vi "TLB Native Dynamic Events ver 0.26a.vi"() -> ()   [LabVIEW 2018] (continued)
              frame "Start Task 1", Default {
                # ">> T: Breaks out of state loop; F: Stays in loop>>"
                # ">> Manual override >>"
                # ">> Checks if time is up>>"
                # "Stays in Task 5D until the object is detected"
                # "T: Go back to idle, F: Continue with task\""
                # ">> Manual override >>"
                n604 = case shown="False" w1776 {
                  tunnel: [w1789 w1795] -> w1785
                  tunnel: w1777 -> [w1787 w1793]
                  frame False {
                    n605 = for {
                      tunnel: string[] ["READ STEPPER VALUES", "Y STEPPER CONTROL", ""] ("element") -> [w1790] mode=indexing
                      shift-right: [w1792] -> w1789
                      shift-left: w1787 -> [w1791]
                      n606 = Enqueue Element(queue=w1791, element=w1790) -> (queue out=w1792:refnum<queue>)  [unwired: 2 in, 2 out]
                    }
                  }
                  frame True {
                    n607 = for {
                      shift-right: [w1797] -> w1795
                      shift-left: w1793 -> [w1798]
                      tunnel: string[] ["DISPOSE BUFFERS", "READ STEPPER VALUES", ""] -> [w1796] mode=indexing
                      n608 = Enqueue Element(queue=w1798, element=w1796) -> (queue out=w1797:refnum<queue>)  [unwired: 2 in, 2 out]
                    }
                  }
                }
                n609 = Or(x=w1776, y=w1781) -> (x .or. y?=w1783:bool)
                n610 = Select(t=State_Type_Definitions,_for_0.26g_versions_and_later_2."True Stop" ("Enum"), s=w1781, f=State_Type_Definitions,_for_0.26g_versions_and_later_2."Task 8I: ARM GRAB HEIGHT" ("Enum")) -> (s? t:f=w1778:T18)
                n611 = Select(t=w1778, s=w1783, f=State_Type_Definitions,_for_0.26g_versions_and_later_2."Task 8H: ARM ADJUST" ("Enum")) -> (s? t:f=w1782:T18)
              }
              frame "Exit" {
                n612 = for {
                  shift-right: [w1805] -> w1802
                  shift-left: w1799 -> [w1806]
                  tunnel: string[] ["STOP", "RESET ENCODERS", "RESET YAW", "ARDUINO MODE 0"] -> [w1804] mode=indexing
                  n613 = Enqueue Element(queue=w1806, element=w1804) -> (queue out=w1805:refnum<queue>)  [unwired: 2 in, 2 out]
                }
              }
            }
            n614 = Bundle By Name(cluster=w1765, "yStepper desired"=w1761) -> (w1764:T20)
          }
          frame 35 {
            # ">>> Motor control cluster >>>"
            # ">>> yStepper command>>>"
            # ">> Manual override >>"
            n615 = Dequeue Element(queue=w1817, timeout in ms (-1)=w1816, error in (no error)=w1818) -> (element=w1815:T10)  [unwired: 3 out]
            n616 = Equal?(x=w1814, y=u8 1) -> (x = y?=w1812:bool)
            n617 = case shown="\"Start Task 1\", Default" w1815 {
              tunnel: [w1828 State_Type_Definitions,_for_0.26g_versions_and_later_2."True Stop" ("Enum")] -> w1819
              tunnel: [w1831 w1848] -> w1820
              tunnel: [State_Type_Definitions,_for_0.26g_versions_and_later_2."Idle" ("Enum") State_Type_Definitions,_for_0.26g_versions_and_later_2."Shutdown" ("Enum")] -> w1821
              tunnel: w1812 -> [w1827 _]
              tunnel: w1811 -> [w1826 _]
              tunnel: w1810 -> [w1822 w1845]
              frame "Start Task 1", Default {
                # "Stays in Task 5F until stepper reaches desired \nheight"
                # "T: Go back to idle, F: Continue with task\""
                # ">> Manual override >>"
                n618 = case shown="True" w1827 {
                  tunnel: [w1835 w1841] -> w1831
                  tunnel: w1822 -> [w1833 w1839]
                  frame False {
                    n619 = for {
                      tunnel: string[] ["Z STEPPER GRAB HEIGHT", "READ STEPPER VALUES"] ("element") -> [w1836] mode=indexing
                      shift-right: [w1838] -> w1835
                      shift-left: w1833 -> [w1837]
                      n620 = Enqueue Element(queue=w1837, element=w1836) -> (queue out=w1838:refnum<queue>)  [unwired: 2 in, 2 out]
                    }
                  }
                  frame True {
                    n621 = for {
                      shift-right: [w1843] -> w1841
                      shift-left: w1839 -> [w1844]
                      tunnel: string[] ["SET TIMER 2", "CLOSE CLAW", ""] -> [w1842] mode=indexing
                      n622 = Enqueue Element(queue=w1844, element=w1842) -> (queue out=w1843:refnum<queue>)  [unwired: 2 in, 2 out]
                    }
                  }
                }
                n623 = Or(x=w1827, y=w1826) -> (x .or. y?=w1829:bool)
                n624 = Select(t=State_Type_Definitions,_for_0.26g_versions_and_later_2."True Stop" ("Enum"), s=w1826, f=State_Type_Definitions,_for_0.26g_versions_and_later_2."Task 8J: CLOSE CLAW" ("Enum")) -> (s? t:f=w1823:T18)
                n625 = Select(t=w1823, s=w1829, f=State_Type_Definitions,_for_0.26g_versions_and_later_2."Task 8I: ARM GRAB HEIGHT" ("Enum")) -> (s? t:f=w1828:T18)
              }
              frame "Exit" {
                n626 = for {
                  shift-right: [w1851] -> w1848
                  shift-left: w1845 -> [w1852]
                  tunnel: string[] ["STOP", "RESET ENCODERS", "RESET YAW", "ARDUINO MODE 0"] -> [w1850] mode=indexing
                  n627 = Enqueue Element(queue=w1852, element=w1850) -> (queue out=w1851:refnum<queue>)  [unwired: 2 in, 2 out]
                }
              }
            }
          }
          frame 36 {
            # ">>> yStepper command>>>"
            # ">> Manual override >>"
            n628 = Dequeue Element(queue=w1863, timeout in ms (-1)=w1862, error in (no error)=w1861) -> (element=w1860:T10)  [unwired: 3 out]
            n629 = case shown="\"Start Task 1\", Default" w1860 {
              tunnel: [w1872 State_Type_Definitions,_for_0.26g_versions_and_later_2."True Stop" ("Enum")] -> w1865
              tunnel: [w1875 w1892] -> w1858
              tunnel: [State_Type_Definitions,_for_0.26g_versions_and_later_2."Idle" ("Enum") State_Type_Definitions,_for_0.26g_versions_and_later_2."Shutdown" ("Enum")] -> w1857
              tunnel: w1859 -> [w1866 _]
              tunnel: w1864 -> [w1871 w1889]
              tunnel: w1855 -> [w1870 _]
              frame "Start Task 1", Default {
                # ">> Is time up? >>"
                # "Determines if object is in range to pick up"
                # ">> Manual override >>"
                n630 = case shown="True" w1870 {
                  tunnel: [w1879 w1885] -> w1875
                  tunnel: w1871 -> [w1877 w1883]
                  frame False {
                    n631 = for {
                      tunnel: string[] ["CLOSE CLAW", "START TIMER"] ("element") -> [w1880] mode=indexing
                      shift-right: [w1882] -> w1879
                      shift-left: w1877 -> [w1881]
                      n632 = Enqueue Element(queue=w1881, element=w1880) -> (queue out=w1882:refnum<queue>)  [unwired: 2 in, 2 out]
                    }
                  }
                  frame True {
                    n633 = for {
                      shift-right: [w1887] -> w1885
                      shift-left: w1883 -> [w1888]
                      tunnel: string[] ["READ STEPPER VALUES", "", ""] -> [w1886] mode=indexing
                      n634 = Enqueue Element(queue=w1888, element=w1886) -> (queue out=w1887:refnum<queue>)  [unwired: 2 in, 2 out]
                    }
                  }
                }
                n635 = Or(x=w1870, y=w1866) -> (x .or. y?=w1873:bool)
                n636 = Select(t=State_Type_Definitions,_for_0.26g_versions_and_later_2."True Stop" ("Enum"), s=w1866, f=State_Type_Definitions,_for_0.26g_versions_and_later_2."Task 8K: RAISE MY SWORD" ("Enum")) -> (s? t:f=w1868:T18)
                n637 = Select(t=w1868, s=w1873, f=State_Type_Definitions,_for_0.26g_versions_and_later_2."Task 8J: CLOSE CLAW" ("Enum")) -> (s? t:f=w1872:T18)
              }
              frame "Exit" {
                n638 = for {
                  shift-right: [w1895] -> w1892
                  shift-left: w1889 -> [w1896]
                  tunnel: string[] ["STOP", "RESET ENCODERS", "RESET YAW", "ARDUINO MODE 0"] -> [w1894] mode=indexing
                  n639 = Enqueue Element(queue=w1896, element=w1894) -> (queue out=w1895:refnum<queue>)  [unwired: 2 in, 2 out]
                }
              }
            }
          }
          frame 37 {
            # ">>> yStepper command>>>"
            # ">> Manual override >>"
            n640 = Dequeue Element(queue=w1907, timeout in ms (-1)=w1906, error in (no error)=w1908) -> (element=w1905:T10)  [unwired: 3 out]
            n641 = Equal?(x=w1904, y=u8 60) -> (x = y?=w1902:bool)
            n642 = case shown="\"Start Task 1\", Default" w1905 {
              tunnel: [w1918 State_Type_Definitions,_for_0.26g_versions_and_later_2."True Stop" ("Enum")] -> w1909
              tunnel: [w1921 w1938] -> w1910
              tunnel: [State_Type_Definitions,_for_0.26g_versions_and_later_2."Idle" ("Enum") State_Type_Definitions,_for_0.26g_versions_and_later_2."Shutdown" ("Enum")] -> w1911
              tunnel: w1902 -> [w1917 _]
              tunnel: w1901 -> [w1916 _]
              tunnel: w1900 -> [w1912 w1935]
              frame "Start Task 1", Default {
                # "Stays in Task 5_A until stepper reaches desired \nheight"
                # "T: Go back to idle, F: Continue with task\""
                # ">> Manual override >>"
                n643 = case shown="True" w1917 {
                  tunnel: [w1925 w1931] -> w1921
                  tunnel: w1912 -> [w1923 w1929]
                  frame False {
                    n644 = for {
                      tunnel: string[] ["Z STEPPER CAM HEIGHT", "READ STEPPER VALUES"] ("element") -> [w1926] mode=indexing
                      shift-right: [w1928] -> w1925
                      shift-left: w1923 -> [w1927]
                      n645 = Enqueue Element(queue=w1927, element=w1926) -> (queue out=w1928:refnum<queue>)  [unwired: 2 in, 2 out]
                    }
                  }
                  frame True {
                    n646 = for {
                      shift-right: [w1933] -> w1931
                      shift-left: w1929 -> [w1934]
                      tunnel: string[] ["CAM CLOSE", "DISPOSE CAM BUFFERS", "DISPOSE PROC BUFFERS", "RESET ENCODERS"] -> [w1932] mode=indexing
                      n647 = Enqueue Element(queue=w1934, element=w1932) -> (queue out=w1933:refnum<queue>)  [unwired: 2 in, 2 out]
                    }
                  }
                }
                n648 = Or(x=w1917, y=w1916) -> (x .or. y?=w1919:bool)
                n649 = Select(t=State_Type_Definitions,_for_0.26g_versions_and_later_2."True Stop" ("Enum"), s=w1916, f=State_Type_Definitions,_for_0.26g_versions_and_later_2."True Stop" ("Enum")) -> (s? t:f=w1913:T18)
                n650 = Select(t=w1913, s=w1919, f=State_Type_Definitions,_for_0.26g_versions_and_later_2."Task 8K: RAISE MY SWORD" ("Enum")) -> (s? t:f=w1918:T18)
              }
              frame "Exit" {
                n651 = for {
                  shift-right: [w1941] -> w1938
                  shift-left: w1935 -> [w1942]
                  tunnel: string[] ["STOP", "RESET ENCODERS", "RESET YAW", "ARDUINO MODE 0"] -> [w1940] mode=indexing
                  n652 = Enqueue Element(queue=w1942, element=w1940) -> (queue out=w1941:refnum<queue>)  [unwired: 2 in, 2 out]
                }
              }
            }
          }
          frame 38 {
            # ">>> Motor control cluster >>>"
            # ">> Stepper height reeached >>"
            # ">>> yStepper command>>>"
            # ">> Manual override >>"
            n653 = Dequeue Element(queue=w1954, timeout in ms (-1)=w1949, error in (no error)=w1953) -> (element=w1957:T10)  [unwired: 3 out]
            n654 = Equal?(x=w1951, y=u8 50) -> (x = y?=w1955:bool)
            n655 = case shown="\"Start Task 1\", Default" w1957 {
              tunnel: [w1968 State_Type_Definitions,_for_0.26g_versions_and_later_2."True Stop" ("Enum")] -> w1947
              tunnel: [w1966 w1983] -> w1946
              tunnel: w1950 -> [w1965 _]
              tunnel: w1952 -> [w1959 _]
              tunnel: [State_Type_Definitions,_for_0.26g_versions_and_later_2."Idle" ("Enum") State_Type_Definitions,_for_0.26g_versions_and_later_2."Shutdown" ("Enum")] -> w1948
              tunnel: w1955 -> [w1958 _]
              frame "Start Task 1", Default {
                # ">> WIill proceed to part ii if not manual override >>"
                # ">>If ENABLE or Trigger is set to true>>"
                n656 = Or(x=w1958, y=w1959) -> (x .or. y?=w1960:bool)
                n657 = case shown="False" w1958 {
                  tunnel: [w1971 w1977] -> w1966
                  tunnel: w1965 -> [w1970 w1976]
                  frame False {
                    n658 = for {
                      shift-right: [w1973] -> w1971
                      shift-left: w1970 -> [w1974]
                      tunnel: string[] ["Z STEPPER BOX HEIGHT", "READ STEPPER VALUES"] ("element") -> [w1972] mode=indexing
                      n659 = Enqueue Element(queue=w1974, element=w1972) -> (queue out=w1973:refnum<queue>)  [unwired: 2 in, 2 out]
                    }
                  }
                  frame True {
                    n660 = for {
                      shift-right: [w1979] -> w1977
                      shift-left: w1976 -> [w1980]
                      tunnel: string[] ["ARDUINO - ULTRASONIC", "READ NAVX", "RESET FLAGS", "", "", ""] -> [w1978] mode=indexing
                      n661 = Enqueue Element(queue=w1980, element=w1978) -> (queue out=w1979:refnum<queue>)  [unwired: 2 in, 2 out]
                    }
                  }
                }
                n662 = Select(t=State_Type_Definitions,_for_0.26g_versions_and_later_2."True Stop" ("Enum"), s=w1959, f=State_Type_Definitions,_for_0.26g_versions_and_later_2."Task 9B: Rotate to Angle" ("Enum")) -> (s? t:f=w1962:T18)
                n663 = Select(t=w1962, s=w1960, f=State_Type_Definitions,_for_0.26g_versions_and_later_2."Task 9A: Raise Arm" ("Enum")) -> (s? t:f=w1968:T18)
              }
              frame "Exit" {
                n664 = for {
                  shift-right: [w1986] -> w1983
                  shift-left: _ -> [w1987]
                  tunnel: string[] ["STOP", "RESET ENCODERS", "RESET YAW", ""] -> [w1985] mode=indexing
                  n665 = Enqueue Element(queue=w1987, element=w1985) -> (queue out=w1986:refnum<queue>)  [unwired: 2 in, 2 out]
                }
              }
            }
          }
          frame 39 {
            # ">>> Motor control cluster >>>"
            # ">>> yStepper command>>>"
            n666 = Dequeue Element(queue=w2001, timeout in ms (-1)=w2000, error in (no error)=w1999) -> (element=w2003:T10)  [unwired: 3 out]
            n667 = In Range and Coerce(upper limit=65.0, x=w1993, lower limit=58.0) -> (In Range?=w1990:bool)  [unwired: 1 out]
            n668 = case shown="\"Start Task 1\", Default" w2003 {
              tunnel: w1994 -> [w2006 _]
              tunnel: [w2014 State_Type_Definitions,_for_0.26g_versions_and_later_2."True Stop" ("Enum")] -> w1996
              tunnel: w2002 -> [w2012 w2030]
              tunnel: [w2011 w2029] -> w1995
              tunnel: [State_Type_Definitions,_for_0.26g_versions_and_later_2."Idle" ("Enum") State_Type_Definitions,_for_0.26g_versions_and_later_2."Shutdown" ("Enum")] -> w1997
              tunnel: w1990 -> [w2004 _]
              frame "Start Task 1", Default {
                n669 = Or(x=w2004, y=w2006) -> (x .or. y?=w2005:bool)
                n670 = case shown="True" w2004 {
                  tunnel: w2012 -> [w2017 w2023]
                  tunnel: [w2016 w2021] -> w2011
                  frame False {
                    n671 = for {
                      shift-right: [w2019] -> w2016
                      shift-left: w2017 -> [w2020]
                      tunnel: string[] ["READ NAVX", "R-CW", "READ ULTRASONIC"] ("element") -> [w2018] mode=indexing
                      n672 = Enqueue Element(queue=w2020, element=w2018) -> (queue out=w2019:refnum<queue>)  [unwired: 2 in, 2 out]
                    }
                  }
                  frame True {
                    n673 = for {
                      shift-right: [w2025] -> w2021
                      shift-left: w2023 -> [w2026]
                      tunnel: string[] ["STOP", "RESET ENCODERS", "RESET YAW", "ARDUINO - ULTRASONIC", ""] -> [w2024] mode=indexing
                      n674 = Enqueue Element(queue=w2026, element=w2024) -> (queue out=w2025:refnum<queue>)  [unwired: 2 in, 2 out]
                    }
                  }
                }
                n675 = Select(t=State_Type_Definitions,_for_0.26g_versions_and_later_2."True Stop" ("Enum"), s=w2006, f=State_Type_Definitions,_for_0.26g_versions_and_later_2."Task 9C: Detect Box") -> (s? t:f=w2008:T18)
                n676 = Select(t=w2008, s=w2005, f=State_Type_Definitions,_for_0.26g_versions_and_later_2."Task 9B: Rotate to Angle" ("Enum")) -> (s? t:f=w2014:T18)
              }
              frame "Exit" {
                n677 = for {
                  shift-right: [w2033] -> w2029
                  shift-left: w2030 -> [w2034]
                  tunnel: string[] ["STOP", "RESET ENCODERS", "RESET YAW", ""] -> [w2032] mode=indexing
                  n678 = Enqueue Element(queue=w2034, element=w2032) -> (queue out=w2033:refnum<queue>)  [unwired: 2 in, 2 out]
                }
              }
            }
          }
          frame 40 {
            # ">>> Motor control cluster >>>"
            # ">>Line Detected>>"
            # ">>Action Queue>>"
            # ">>> yStepper command>>>"
            n679 = Dequeue Element(queue=w2046, timeout in ms (-1)=w2045, error in (no error)=w2044) -> (element=w2047:T10)  [unwired: 3 out]
            n680 = case shown="\"Start Task 1\", Default" w2047 {
              tunnel: w2042 -> [w2048 _]
              tunnel: [w2058 State_Type_Definitions,_for_0.26g_versions_and_later_2."True Stop" ("Enum")] -> w2039
              tunnel: w2043 -> [w2056 w2074]
              tunnel: [w2055 w2073] -> w2038
              tunnel: [State_Type_Definitions,_for_0.26g_versions_and_later_2."Idle" ("Enum") State_Type_Definitions,_for_0.26g_versions_and_later_2."Shutdown" ("Enum")] -> w2041
              tunnel: w2036 -> [w2049 _]
              frame "Start Task 1", Default {
                n681 = Or(x=w2048, y=w2049) -> (x .or. y?=w2050:bool)
                n682 = case shown="True" w2049 {
                  tunnel: w2056 -> [w2061 w2067]
                  tunnel: [w2060 w2065] -> w2055
                  frame False {
                    n683 = for {
                      shift-right: [w2063] -> w2060
                      shift-left: w2061 -> [w2064]
                      tunnel: string[] ["READ IR", "READ LINE SENSOR", "FORWARD - IR ASSIST"] ("element") -> [w2062] mode=indexing
                      n684 = Enqueue Element(queue=w2064, element=w2062) -> (queue out=w2063:refnum<queue>)  [unwired: 2 in, 2 out]
                    }
                  }
                  frame True {
                    n685 = for {
                      shift-right: [w2069] -> w2065
                      shift-left: w2067 -> [w2070]
                      tunnel: string[] ["STOP", "RESET ENCODERS", "RESET YAW", ""] -> [w2068] mode=indexing
                      n686 = Enqueue Element(queue=w2070, element=w2068) -> (queue out=w2069:refnum<queue>)  [unwired: 2 in, 2 out]
                    }
                  }
                }
                n687 = Select(t=State_Type_Definitions,_for_0.26g_versions_and_later_2."True Stop" ("Enum"), s=w2048, f=State_Type_Definitions,_for_0.26g_versions_and_later_2."Task 9D: MOVE FORWARD") -> (s? t:f=w2052:T18)
                n688 = Select(t=w2052, s=w2050, f=State_Type_Definitions,_for_0.26g_versions_and_later_2."Task 9C: Detect Box" ("Enum")) -> (s? t:f=w2058:T18)
              }
              frame "Exit" {
                n689 = for {
                  shift-right: [w2077] -> w2073
                  shift-left: w2074 -> [w2078]
                  tunnel: string[] ["STOP", "RESET ENCODERS", "RESET YAW", ""] -> [w2076] mode=indexing
                  n690 = Enqueue Element(queue=w2078, element=w2076) -> (queue out=w2077:refnum<queue>)  [unwired: 2 in, 2 out]
                }
              }
            }
          }
          frame 41 {
            (unwired) 50.0 ("y")
            # ">> Item Selection Bias >>"
            # ">> Wall detected >>"
            # ">> Manual override >>"
            # ">>Table Detected>>"
            # ">>> Motor control cluster >>>"
            # ">>Table or wall detectected>>"
            # ">>Action Queue>>"
            # ">>> yStepper command>>>"
            n691 = Dequeue Element(queue=w2097, timeout in ms (-1)=w2096, error in (no error)=w2095) -> (element=w2098:T10)  [unwired: 3 out]
            n692 = Less Or Equal?(x=w2086, y=15.0) -> (x <= y?=w2081:bool)
            n693 = Less?(x=w2084, y=20.0) -> (x < y?=w2082:bool)
            n694 = Or(x=w2081, y=w2082) -> (x .or. y?=w2079:bool)
            n695 = And(x=w2079, y=w2079) -> (x .and. y?=w2080:bool)
            n696 = case shown="\"Start Task 1\", Default" w2098 {
              tunnel: w2093 -> [w2099 _]
              tunnel: [w2109 State_Type_Definitions,_for_0.26g_versions_and_later_2."True Stop" ("Enum")] -> w2090
              tunnel: w2094 -> [w2107 w2125]
              tunnel: [w2106 w2124] -> w2089
              tunnel: [State_Type_Definitions,_for_0.26g_versions_and_later_2."Idle" ("Enum") State_Type_Definitions,_for_0.26g_versions_and_later_2."Shutdown" ("Enum")] -> w2092
              tunnel: w2080 -> [w2100 _]
              frame "Start Task 1", Default {
                n697 = Or(x=w2099, y=w2100) -> (x .or. y?=w2101:bool)
                n698 = case shown="False" w2100 {
                  tunnel: w2107 -> [w2112 w2118]
                  tunnel: [w2111 w2116] -> w2106
                  frame False {
                    n699 = for {
                      shift-right: [w2114] -> w2111
                      shift-left: w2112 -> [w2115]
                      tunnel: string[] ["READ IR", "FORWARD - IR ASSIST", "READ ULTRASONIC"] ("element") -> [w2113] mode=indexing
                      n700 = Enqueue Element(queue=w2115, element=w2113) -> (queue out=w2114:refnum<queue>)  [unwired: 2 in, 2 out]
                    }
                  }
                  frame True {
                    n701 = for {
                      shift-right: [w2120] -> w2116
                      shift-left: w2118 -> [w2121]
                      tunnel: string[] ["STOP", "RESET ENCODERS", "RESET YAW", ""] -> [w2119] mode=indexing
                      n702 = Enqueue Element(queue=w2121, element=w2119) -> (queue out=w2120:refnum<queue>)  [unwired: 2 in, 2 out]
                    }
                  }
                }
                n703 = Select(t=State_Type_Definitions,_for_0.26g_versions_and_later_2."True Stop" ("Enum"), s=w2099, f=State_Type_Definitions,_for_0.26g_versions_and_later_2."Task 9E: MOVE LEFT") -> (s? t:f=w2103:T18)
                n704 = Select(t=w2103, s=w2101, f=State_Type_Definitions,_for_0.26g_versions_and_later_2."Task 9D: MOVE FORWARD" ("Enum")) -> (s? t:f=w2109:T18)
              }
              frame "Exit" {
                n705 = for {
                  shift-right: [w2128] -> w2124
                  shift-left: w2125 -> [w2129]
                  tunnel: string[] ["STOP", "RESET ENCODERS", "RESET YAW", ""] -> [w2127] mode=indexing
                  n706 = Enqueue Element(queue=w2129, element=w2127) -> (queue out=w2128:refnum<queue>)  [unwired: 2 in, 2 out]
                }
              }
            }
          }
          frame 42 {
            # ">> Item Selection Bias >>"
            # ">> Line detected? >>"
            # ">> Manual override >>"
            # ">>> Motor control cluster >>>"
            # ">>Action Queue>>"
            # ">>> yStepper command>>>"
            n707 = Dequeue Element(queue=w2141, timeout in ms (-1)=w2140, error in (no error)=w2139) -> (element=w2142:T10)  [unwired: 3 out]
            n708 = case shown="\"Start Task 1\", Default" w2142 {
              tunnel: w2137 -> [w2143 _]
              tunnel: [w2153 State_Type_Definitions,_for_0.26g_versions_and_later_2."True Stop" ("Enum")] -> w2134
              tunnel: w2138 -> [w2151 w2169]
              tunnel: [w2150 w2168] -> w2133
              tunnel: [State_Type_Definitions,_for_0.26g_versions_and_later_2."Idle" ("Enum") State_Type_Definitions,_for_0.26g_versions_and_later_2."Shutdown" ("Enum")] -> w2136
              tunnel: w2130 -> [w2144 _]
              frame "Start Task 1", Default {
                n709 = Or(x=w2143, y=w2144) -> (x .or. y?=w2145:bool)
                n710 = case shown="False" w2144 {
                  tunnel: w2151 -> [w2156 w2162]
                  tunnel: [w2155 w2160] -> w2150
                  frame False {
                    n711 = for {
                      shift-right: [w2158] -> w2155
                      shift-left: w2156 -> [w2159]
                      tunnel: string[] ["LEFT", "READ NAVX", "READ LINE SENSOR", ""] ("element") -> [w2157] mode=indexing
                      n712 = Enqueue Element(queue=w2159, element=w2157) -> (queue out=w2158:refnum<queue>)  [unwired: 2 in, 2 out]
                    }
                  }
                  frame True {
                    n713 = for {
                      shift-right: [w2164] -> w2160
                      shift-left: w2162 -> [w2165]
                      tunnel: string[] ["STOP", "RESET ENCODERS", "RESET YAW", "RESET FLAGS", "OPEN LIFE CAM", "SET TIMER 2"] -> [w2163] mode=indexing
                      n714 = Enqueue Element(queue=w2165, element=w2163) -> (queue out=w2164:refnum<queue>)  [unwired: 2 in, 2 out]
                    }
                  }
                }
                n715 = Select(t=State_Type_Definitions,_for_0.26g_versions_and_later_2."True Stop" ("Enum"), s=w2143, f=State_Type_Definitions."Task 9F: SCAN IMAGE") -> (s? t:f=w2147:u16)
                n716 = Select(t=w2147, s=w2145, f=State_Type_Definitions,_for_0.26g_versions_and_later_2."Task 9E: MOVE LEFT" ("Enum")) -> (s? t:f=w2153:u16)
              }
              frame "Exit" {
                n717 = for {
                  shift-right: [w2172] -> w2168
                  shift-left: w2169 -> [w2173]
                  tunnel: string[] ["STOP", "RESET ENCODERS", "RESET YAW", ""] -> [w2171] mode=indexing
                  n718 = Enqueue Element(queue=w2173, element=w2171) -> (queue out=w2172:refnum<queue>)  [unwired: 2 in, 2 out]
                }
              }
            }
          }
          frame 43 {
            # ">>> Motor control cluster >>>"
            # ">>Time up? >>"
            # ">>> yStepper command>>>"
            # ">> Manual override >>"
            n719 = Dequeue Element(queue=w2185, timeout in ms (-1)=w2181, error in (no error)=w2184) -> (element=w2186:T10)  [unwired: 3 out]
            n720 = case shown="\"Start Task 1\", Default" w2186 {
              tunnel: [w2197 State_Type_Definitions,_for_0.26g_versions_and_later_2."True Stop" ("Enum")] -> w2179
              tunnel: [w2195 w2213] -> w2178
              tunnel: w2182 -> [w2194 w2210]
              tunnel: w2183 -> [w2188 _]
              tunnel: [State_Type_Definitions,_for_0.26g_versions_and_later_2."Idle" ("Enum") State_Type_Definitions,_for_0.26g_versions_and_later_2."Shutdown" ("Enum")] -> w2180
              tunnel: w2174 -> [w2187 _]
              frame "Start Task 1", Default {
                # ">> WIill proceed to part ii if not manual override >>"
                # ">>If ENABLE or Trigger is set to true>>"
                n721 = Or(x=w2187, y=w2188) -> (x .or. y?=w2189:bool)
                n722 = case shown="True" w2187 {
                  tunnel: [w2200 w2206] -> w2195
                  tunnel: w2194 -> [w2199 w2205]
                  frame False {
                    n723 = for {
                      shift-right: [w2202] -> w2200
                      shift-left: w2199 -> [w2203]
                      tunnel: string[] ["CAM ACQ", "START TIMER"] ("element") -> [w2201] mode=indexing
                      n724 = Enqueue Element(queue=w2203, element=w2201) -> (queue out=w2202:refnum<queue>)  [unwired: 2 in, 2 out]
                    }
                  }
                  frame True {
                    n725 = for {
                      shift-right: [w2208] -> w2206
                      shift-left: w2205 -> [w2209]
                      tunnel: string[] ["CLOSE CAM", "SET TIMER 5", "", "", "", ""] -> [w2207] mode=indexing
                      n726 = Enqueue Element(queue=w2209, element=w2207) -> (queue out=w2208:refnum<queue>)  [unwired: 2 in, 2 out]
                    }
                  }
                }
                n727 = Select(t=State_Type_Definitions,_for_0.26g_versions_and_later_2."True Stop" ("Enum"), s=w2188, f=State_Type_Definitions."Task 9G: PROCESS COLOUR" ("Enum")) -> (s? t:f=w2191:u16)
                n728 = Select(t=w2191, s=w2189, f=State_Type_Definitions."Task 9F: SCAN IMAGE" ("Enum")) -> (s? t:f=w2197:u16)
              }
              frame "Exit" {
                n729 = for {
                  shift-right: [w2216] -> w2213
                  shift-left: w2210 -> [w2217]
                  tunnel: string[] ["STOP", "RESET ENCODERS", "RESET YAW", ""] -> [w2215] mode=indexing
                  n730 = Enqueue Element(queue=w2217, element=w2215) -> (queue out=w2216:refnum<queue>)  [unwired: 2 in, 2 out]
                }
              }
            }
          }
          frame 44 {
            # ">>> Motor control cluster >>>"
            # ">>> yStepper command>>>"
            n731 = Dequeue Element(queue=w2225, timeout in ms (-1)=w2224, error in (no error)=w2223) -> (element=w2230:T10)  [unwired: 3 out]
            n732 = case shown="\"Start Task 1\", Default" w2230 {
              tunnel: w2218 -> [w2233 _]
              tunnel: [w2240 State_Type_Definitions,_for_0.26g_versions_and_later_2."True Stop" ("Enum")] -> w2229
              tunnel: w2222 -> [w2232 _]
              tunnel: w2226 -> [w2239 w2256]
              tunnel: [w2238 w2257] -> w2228
              tunnel: [State_Type_Definitions,_for_0.26g_versions_and_later_2."Idle" ("Enum") State_Type_Definitions,_for_0.26g_versions_and_later_2."Shutdown" ("Enum")] -> w2227
              frame "Start Task 1", Default {
                n733 = case shown="False" w2233 {
                  tunnel: w2239 -> [w2243 w2250]
                  tunnel: [w2244 w2249] -> w2238
                  frame False {
                    n734 = for {
                      tunnel: string[] ["START TIMER", "COLOUR PROCESSING", ""] ("element") -> [w2245] mode=indexing
                      shift-right: [w2247] -> w2244
                      shift-left: w2243 -> [w2246]
                      n735 = Enqueue Element(queue=w2246, element=w2245) -> (queue out=w2247:refnum<queue>)  [unwired: 2 in, 2 out]
                    }
                  }
                  frame True {
                    n736 = for {
                      shift-right: [w2252] -> w2249
                      shift-left: w2250 -> [w2253]
                      tunnel: string[] ["DISPOSE BUFFERS", "CLOSE CAM", "RESET ENCODERS", "RESET YAW", "RESET FLAGS"] -> [w2251] mode=indexing
                      n737 = Enqueue Element(queue=w2253, element=w2251) -> (queue out=w2252:refnum<queue>)  [unwired: 2 in, 2 out]
                    }
                  }
                }
                n738 = Or(x=w2233, y=w2232) -> (x .or. y?=w2231:bool)
                n739 = Select(t=State_Type_Definitions,_for_0.26g_versions_and_later_2."True Stop" ("Enum"), s=w2232, f=State_Type_Definitions,_for_0.26g_versions_and_later_2."True Stop" ("Enum")) -> (s? t:f=w2234:T18)
                n740 = Select(t=w2234, s=w2231, f=State_Type_Definitions."Task 9G: PROCESS COLOUR" ("Enum")) -> (s? t:f=w2240:u16)
              }
              frame "Exit" {
                n741 = for {
                  shift-right: [w2260] -> w2257
                  shift-left: w2256 -> [w2261]
                  tunnel: string[] ["STOP", "RESET ENCODERS", "RESET YAW", "ARDUINO MODE 0"] -> [w2259] mode=indexing
                  n742 = Enqueue Element(queue=w2261, element=w2259) -> (queue out=w2260:refnum<queue>)  [unwired: 2 in, 2 out]
                }
              }
            }
          }
          frame 45 {
            # ">> Item Selection Bias >>"
            # ">>> Motor control cluster >>>"
            # ">>> yStepper command>>>"
            n743 = Dequeue Element(queue=w2271, timeout in ms (-1)=w2272, error in (no error)=w2273) -> (element=w2275:T10)  [unwired: 3 out]
            n744 = Greater?(x=w2263, y=50.0) -> (0:w2264:bool)
            n745 = And(x=w2265, y=w2264) -> (x .and. y?=w2266:bool)
            n746 = case shown="\"Start Task 1\", Default" w2275 {
              tunnel: w2266 -> [w2281 _]
              tunnel: [w2288 State_Type_Definitions,_for_0.26g_versions_and_later_2."True Stop" ("Enum")] -> w2268
              tunnel: w2274 -> [w2280 _]
              tunnel: w2270 -> [w2287 w2304]
              tunnel: [w2286 w2305] -> w2269
              tunnel: [State_Type_Definitions,_for_0.26g_versions_and_later_2."Idle" ("Enum") State_Type_Definitions,_for_0.26g_versions_and_later_2."Shutdown" ("Enum")] -> w2267
              frame "Start Task 1", Default {
                n747 = case shown="True" w2281 {
                  tunnel: w2287 -> [w2291 w2298]
                  tunnel: [w2292 w2297] -> w2286
                  frame False {
                    n748 = for {
                      tunnel: string[] ["READ LINE SENSOR", "READ NAVX", "RIGHT", "READ ENCODERS"] ("element") -> [w2293] mode=indexing
                      shift-right: [w2295] -> w2292
                      shift-left: w2291 -> [w2294]
                      n749 = Enqueue Element(queue=w2294, element=w2293) -> (queue out=w2295:refnum<queue>)  [unwired: 2 in, 2 out]
                    }
                  }
                  frame True {
                    n750 = for {
                      shift-right: [w2300] -> w2297
                      shift-left: w2298 -> [w2301]
                      tunnel: string[] ["STOP", "RESET ENCODERS", "RESET YAW", "OPEN LIFE CAM", "SET TIMER 5", "RESET FLAGS"] -> [w2299] mode=indexing
                      n751 = Enqueue Element(queue=w2301, element=w2299) -> (queue out=w2300:refnum<queue>)  [unwired: 2 in, 2 out]
                    }
                  }
                }
                n752 = Or(x=w2281, y=w2280) -> (x .or. y?=w2279:bool)
                n753 = Select(t=State_Type_Definitions,_for_0.26g_versions_and_later_2."True Stop" ("Enum"), s=w2280, f=State_Type_Definitions,_for_0.26d_versions_and_later."Task 9I: SCAN IMAGE" ("Enum")) -> (s? t:f=w2282:u16)
                n754 = Select(t=w2282, s=w2279, f=State_Type_Definitions."Task 9H: MOVE RIGHT" ("Enum")) -> (s? t:f=w2288:u16)
              }
              frame "Exit" {
                n755 = for {
                  shift-right: [w2308] -> w2305
                  shift-left: w2304 -> [w2309]
                  tunnel: string[] ["STOP", "RESET ENCODERS", "RESET YAW", "ARDUINO MODE 0"] -> [w2307] mode=indexing
                  n756 = Enqueue Element(queue=w2309, element=w2307) -> (queue out=w2308:refnum<queue>)  [unwired: 2 in, 2 out]
                }
              }
            }
          }
          frame 46 {
            # ">> Item Selection Bias >>"
            n757 = Dequeue Element(queue=w2311, timeout in ms (-1)=w2312, error in (no error)=w2313) -> (element=w2319:T10)  [unwired: 3 out]
            n758 = case shown="\"Start Task 1\", Default" w2319 {
              tunnel: w2310 -> [w2325 _]
              tunnel: [w2332 State_Type_Definitions,_for_0.26g_versions_and_later_2."True Stop" ("Enum")] -> w2316
              tunnel: w2314 -> [w2324 _]
              tunnel: w2318 -> [w2331 w2348]
              tunnel: [w2330 w2349] -> w2317
              tunnel: [State_Type_Definitions,_for_0.26g_versions_and_later_2."Idle" ("Enum") State_Type_Definitions,_for_0.26g_versions_and_later_2."Shutdown" ("Enum")] -> w2315
              frame "Start Task 1", Default {
                n759 = case shown="True" w2325 {
                  tunnel: w2331 -> [w2335 w2342]
                  tunnel: [w2336 w2341] -> w2330
                  frame False {
                    n760 = for {
                      tunnel: string[] ["START TIMER", "CAM ACQ", ""] ("element") -> [w2337] mode=indexing
                      shift-right: [w2339] -> w2336
                      shift-left: w2335 -> [w2338]
                      n761 = Enqueue Element(queue=w2338, element=w2337) -> (queue out=w2339:refnum<queue>)  [unwired: 2 in, 2 out]
                    }
                  }
                  frame True {
                    n762 = for {
                      shift-right: [w2344] -> w2341
                      shift-left: w2342 -> [w2345]
                      tunnel: string[] ["CLOSE CAM", "SET TIMER 5", "", "", "", ""] -> [w2343] mode=indexing
                      n763 = Enqueue Element(queue=w2345, element=w2343) -> (queue out=w2344:refnum<queue>)  [unwired: 2 in, 2 out]
                    }
                  }
                }
                n764 = Or(x=w2325, y=w2324) -> (x .or. y?=w2323:bool)
                n765 = Select(t=State_Type_Definitions,_for_0.26g_versions_and_later_2."True Stop" ("Enum"), s=w2324, f=State_Type_Definitions,_for_0.26d_versions_and_later."Task 9J: PROCESS COLOUR" ("Enum")) -> (s? t:f=w2326:u16)
                n766 = Select(t=w2326, s=w2323, f=State_Type_Definitions,_for_0.26d_versions_and_later."Task 9I: SCAN IMAGE" ("Enum")) -> (s? t:f=w2332:u16)
              }
              frame "Exit" {
                n767 = for {
                  shift-right: [w2352] -> w2349
                  shift-left: w2348 -> [w2353]
                  tunnel: string[] ["STOP", "RESET ENCODERS", "RESET YAW", "ARDUINO MODE 0"] -> [w2351] mode=indexing
                  n768 = Enqueue Element(queue=w2353, element=w2351) -> (queue out=w2352:refnum<queue>)  [unwired: 2 in, 2 out]
                }
              }
            }
          }
          frame 47 {
            # ">> Item Selection Bias >>"
            n769 = Dequeue Element(queue=w2359, timeout in ms (-1)=w2360, error in (no error)=w2361) -> (element=w2363:T10)  [unwired: 3 out]
            n770 = case shown="\"Start Task 1\", Default" w2363 {
              tunnel: w2354 -> [w2369 _]
              tunnel: [w2376 State_Type_Definitions,_for_0.26g_versions_and_later_2."True Stop" ("Enum")] -> w2357
              tunnel: w2362 -> [w2368 _]
              tunnel: w2358 -> [w2375 w2392]
              tunnel: [w2374 w2393] -> w2356
              tunnel: [State_Type_Definitions,_for_0.26g_versions_and_later_2."Idle" ("Enum") State_Type_Definitions,_for_0.26g_versions_and_later_2."Shutdown" ("Enum")] -> w2355
              frame "Start Task 1", Default {
                n771 = case shown="True" w2369 {
                  tunnel: w2375 -> [w2379 w2386]
                  tunnel: [w2380 w2385] -> w2374
                  frame False {
                    n772 = for {
                      tunnel: string[] ["START TIMER", "COLOUR PROCESSING", ""] ("element") -> [w2381] mode=indexing
                      shift-right: [w2383] -> w2380
                      shift-left: w2379 -> [w2382]
                      n773 = Enqueue Element(queue=w2382, element=w2381) -> (queue out=w2383:refnum<queue>)  [unwired: 2 in, 2 out]
                    }
                  }
                  frame True {
                    n774 = for {
                      shift-right: [w2388] -> w2385
                      shift-left: w2386 -> [w2389]
                      tunnel: string[] ["CLOSE CAM", "DISPOSE BUFFERS", "RESET ENCODERS", "RESET YAW", "RESET FLAGS", ""] -> [w2387] mode=indexing
                      n775 = Enqueue Element(queue=w2389, element=w2387) -> (queue out=w2388:refnum<queue>)  [unwired: 2 in, 2 out]
                    }
                  }
                }
                n776 = Or(x=w2369, y=w2368) -> (x .or. y?=w2367:bool)
                n777 = Select(t=State_Type_Definitions,_for_0.26g_versions_and_later_2."True Stop" ("Enum"), s=w2368, f=State_Type_Definitions,_for_0.26g_versions_and_later_2."True Stop" ("Enum")) -> (s? t:f=w2370:T18)
                n778 = Select(t=w2370, s=w2367, f=State_Type_Definitions,_for_0.26d_versions_and_later."Task 9J: PROCESS COLOUR" ("Enum")) -> (s? t:f=w2376:u16)
              }
              frame "Exit" {
                n779 = for {
                  shift-right: [w2396] -> w2393
                  shift-left: w2392 -> [w2397]
                  tunnel: string[] ["STOP", "RESET ENCODERS", "RESET YAW", "ARDUINO MODE 0"] -> [w2395] mode=indexing
                  n780 = Enqueue Element(queue=w2397, element=w2395) -> (queue out=w2396:refnum<queue>)  [unwired: 2 in, 2 out]
                }
              }
            }
          }
          frame 48 {
            # ">>> Motor control cluster >>>"
            # ">>> yStepper command>>>"
            # ">> Item Selection Bias >>"
            n781 = Less?(x=w2401, y=-38.0) -> (x < y?=w2399:bool)
            n782 = Dequeue Element(queue=w2407, timeout in ms (-1)=w2406, error in (no error)=w2405) -> (element=w2409:T10)  [unwired: 3 out]
            n783 = case shown="\"Start Task 1\", Default" w2409 {
              tunnel: w2399 -> [w2415 _]
              tunnel: [w2422 State_Type_Definitions,_for_0.26g_versions_and_later_2."True Stop" ("Enum")] -> w2403
              tunnel: w2404 -> [w2414 _]
              tunnel: w2408 -> [w2421 w2438]
              tunnel: [w2420 w2439] -> w2398
              tunnel: [State_Type_Definitions,_for_0.26g_versions_and_later_2."Idle" ("Enum") State_Type_Definitions,_for_0.26g_versions_and_later_2."Shutdown" ("Enum")] -> w2402
              frame "Start Task 1", Default {
                n784 = case shown="True" w2415 {
                  tunnel: w2421 -> [w2425 w2432]
                  tunnel: [w2426 w2431] -> w2420
                  frame False {
                    n785 = for {
                      tunnel: string[] ["READ ENCODERS", "R-CW"] ("element") -> [w2427] mode=indexing
                      shift-right: [w2429] -> w2426
                      shift-left: w2425 -> [w2428]
                      n786 = Enqueue Element(queue=w2428, element=w2427) -> (queue out=w2429:refnum<queue>)  [unwired: 2 in, 2 out]
                    }
                  }
                  frame True {
                    n787 = for {
                      shift-right: [w2434] -> w2431
                      shift-left: w2432 -> [w2435]
                      tunnel: string[] ["STOP", "RESET ENCODERS", "RESET FLAGS", "RESET YAW", "READ IR", "ARDUINO - ULTRASONIC"] -> [w2433] mode=indexing
                      n788 = Enqueue Element(queue=w2435, element=w2433) -> (queue out=w2434:refnum<queue>)  [unwired: 2 in, 2 out]
                    }
                  }
                }
                n789 = Or(x=w2415, y=w2414) -> (x .or. y?=w2413:bool)
                n790 = Select(t=State_Type_Definitions,_for_0.26g_versions_and_later_2."True Stop" ("Enum"), s=w2414, f=State_Type_Definitions,_for_0.26d_versions_and_later."Task 9L: MOVE FORWARD" ("Enum")) -> (s? t:f=w2416:u16)
                n791 = Select(t=w2416, s=w2413, f=State_Type_Definitions,_for_0.26d_versions_and_later."Task 9K: ROTATE 90 CW" ("Enum")) -> (s? t:f=w2422:u16)
              }
              frame "Exit" {
                n792 = for {
                  shift-right: [w2442] -> w2439
                  shift-left: w2438 -> [w2443]
                  tunnel: string[] ["STOP", "RESET ENCODERS", "RESET YAW", "ARDUINO MODE 0"] -> [w2441] mode=indexing
                  n793 = Enqueue Element(queue=w2443, element=w2441) -> (queue out=w2442:refnum<queue>)  [unwired: 2 in, 2 out]
                }
              }
            }
          }
          frame 49 {
            w2456 = u8 50 ("y")
            # ">>> Motor control cluster >>>"
            # ">>> yStepper command>>>"
            # ">> Item Selection Bias >>"
            n794 = Less?(x=w2458, y=w2456) -> (x < y?=w2451:bool)
            n795 = Dequeue Element(queue=w2462, timeout in ms (-1)=w2461, error in (no error)=w2460) -> (element=w2466:T10)  [unwired: 3 out]
            n796 = Less?(x=w2457, y=w2456) -> (x < y?=w2452:bool)
            n797 = And(x=w2452, y=w2451) -> (x .and. y?=w2444:bool)
            n798 = Less Or Equal?(x=w2455, y=15.0) -> (x <= y?=w2450:bool)
            n799 = Greater?(x=w2449, y=100.0) -> (0:w2448:bool)
            n800 = Or(x=w2450, y=w2444) -> (x .or. y?=w2446:bool)
            n801 = And(x=w2448, y=w2446) -> (x .and. y?=w2447:bool)
            n802 = case shown="\"Start Task 1\", Default" w2466 {
              tunnel: w2447 -> [w2472 _]
              tunnel: [w2479 State_Type_Definitions,_for_0.26g_versions_and_later_2."True Stop" ("Enum")] -> w2464
              tunnel: w2459 -> [w2471 _]
              tunnel: w2463 -> [w2478 w2495]
              tunnel: [w2477 w2496] -> w2453
              tunnel: [State_Type_Definitions,_for_0.26g_versions_and_later_2."Idle" ("Enum") State_Type_Definitions,_for_0.26g_versions_and_later_2."Shutdown" ("Enum")] -> w2465
              frame "Start Task 1", Default {
                n803 = case shown="True" w2472 {
                  tunnel: w2478 -> [w2482 w2489]
                  tunnel: [w2483 w2488] -> w2477
                  frame False {
                    n804 = for {
                      tunnel: string[] ["READ IR", "FORWARD", "READ NAVX", "READ ENCODERS"] ("element") -> [w2484] mode=indexing
                      shift-right: [w2486] -> w2483
                      shift-left: w2482 -> [w2485]
                      n805 = Enqueue Element(queue=w2485, element=w2484) -> (queue out=w2486:refnum<queue>)  [unwired: 2 in, 2 out]
                    }
                  }
                  frame True {
                    n806 = for {
                      shift-right: [w2491] -> w2488
                      shift-left: w2489 -> [w2492]
                      tunnel: string[] ["STOP", "RESET ENCODERS", "RESET FLAGS", "RESET YAW", "", ""] -> [w2490] mode=indexing
                      n807 = Enqueue Element(queue=w2492, element=w2490) -> (queue out=w2491:refnum<queue>)  [unwired: 2 in, 2 out]
                    }
                  }
                }
                n808 = Or(x=w2472, y=w2471) -> (x .or. y?=w2470:bool)
                n809 = Select(t=State_Type_Definitions,_for_0.26g_versions_and_later_2."True Stop" ("Enum"), s=w2471, f=State_Type_Definitions,_for_0.26g_versions_and_later_2."True Stop" ("Enum")) -> (s? t:f=w2473:T18)
                n810 = Select(t=w2473, s=w2470, f=State_Type_Definitions,_for_0.26d_versions_and_later."Task 9L: MOVE FORWARD" ("Enum")) -> (s? t:f=w2479:u16)
              }
              frame "Exit" {
                n811 = for {
                  shift-right: [w2499] -> w2496
                  shift-left: w2495 -> [w2500]
                  tunnel: string[] ["STOP", "RESET ENCODERS", "RESET YAW", "ARDUINO MODE 0"] -> [w2498] mode=indexing
                  n812 = Enqueue Element(queue=w2500, element=w2498) -> (queue out=w2499:refnum<queue>)  [unwired: 2 in, 2 out]
                }
              }
            }
          }
          frame 50 {
            # ">> Item Selection Bias >>"
            n813 = Dequeue Element(queue=w2505, timeout in ms (-1)=w2504, error in (no error)=w2503) -> (element=w2510:T10)  [unwired: 3 out]
            n814 = case shown="\"Start Task 1\", Default" w2510 {
              tunnel: w2501 -> [w2516 _]
              tunnel: [w2523 State_Type_Definitions,_for_0.26g_versions_and_later_2."True Stop" ("Enum")] -> w2508
              tunnel: w2502 -> [w2515 _]
              tunnel: w2506 -> [w2522 w2539]
              tunnel: [w2521 w2540] -> w2507
              tunnel: [State_Type_Definitions,_for_0.26g_versions_and_later_2."Idle" ("Enum") State_Type_Definitions,_for_0.26g_versions_and_later_2."Shutdown" ("Enum")] -> w2509